vi "Main.vi"() -> ()   [LabVIEW 2020]
uses:
  Global_Variable/Global.vi
  Database/Global1.vi
  <userlib>/_MGI/Menu Building/MenuTypes/MenuStrip/MGI_MenuStrip.lvclass
  Libraries/S7/S7.lvlib
  <userlib>/_MGI/Menu Building/MenuItemStatusChange/MGI_MenuItemStatusChange.lvclass
  System.Windows.Forms
panel:
  in  "VI引用句柄":refnum<vi>
  out "结果显示:":string
  out "传感器值":dbl format="%#_4gN"
  in  "打印条码":bool caption="布尔"
  out "自动":bool
  out "管柱码":string
  out "上序状态":string
  in  "Andon":enum32{"未选择", "缺料报警", "质量报警", "故障报警"}(radio)
  out "PLC":bool
  in  "菜单":refnum<k24>(container)
  in  "Result":string[][](table)
  out "试验计时":u16 format="%.0fS"
  out "生产数量":i32 format="%.0f件"
  out "合格数量":i32 format="%.0f件"
  out "userStatus":string caption="用户状态"
  out "userName":string caption="用户名"
  out "connectionMode":string caption="联机类型"
  out "产品型号":string
  out "锁紧/开启":bool
  out "提示信息":string
  out "错误":bool
  out "时间字符串":string
  out "日期字符串":string
  # "中间轴装配"
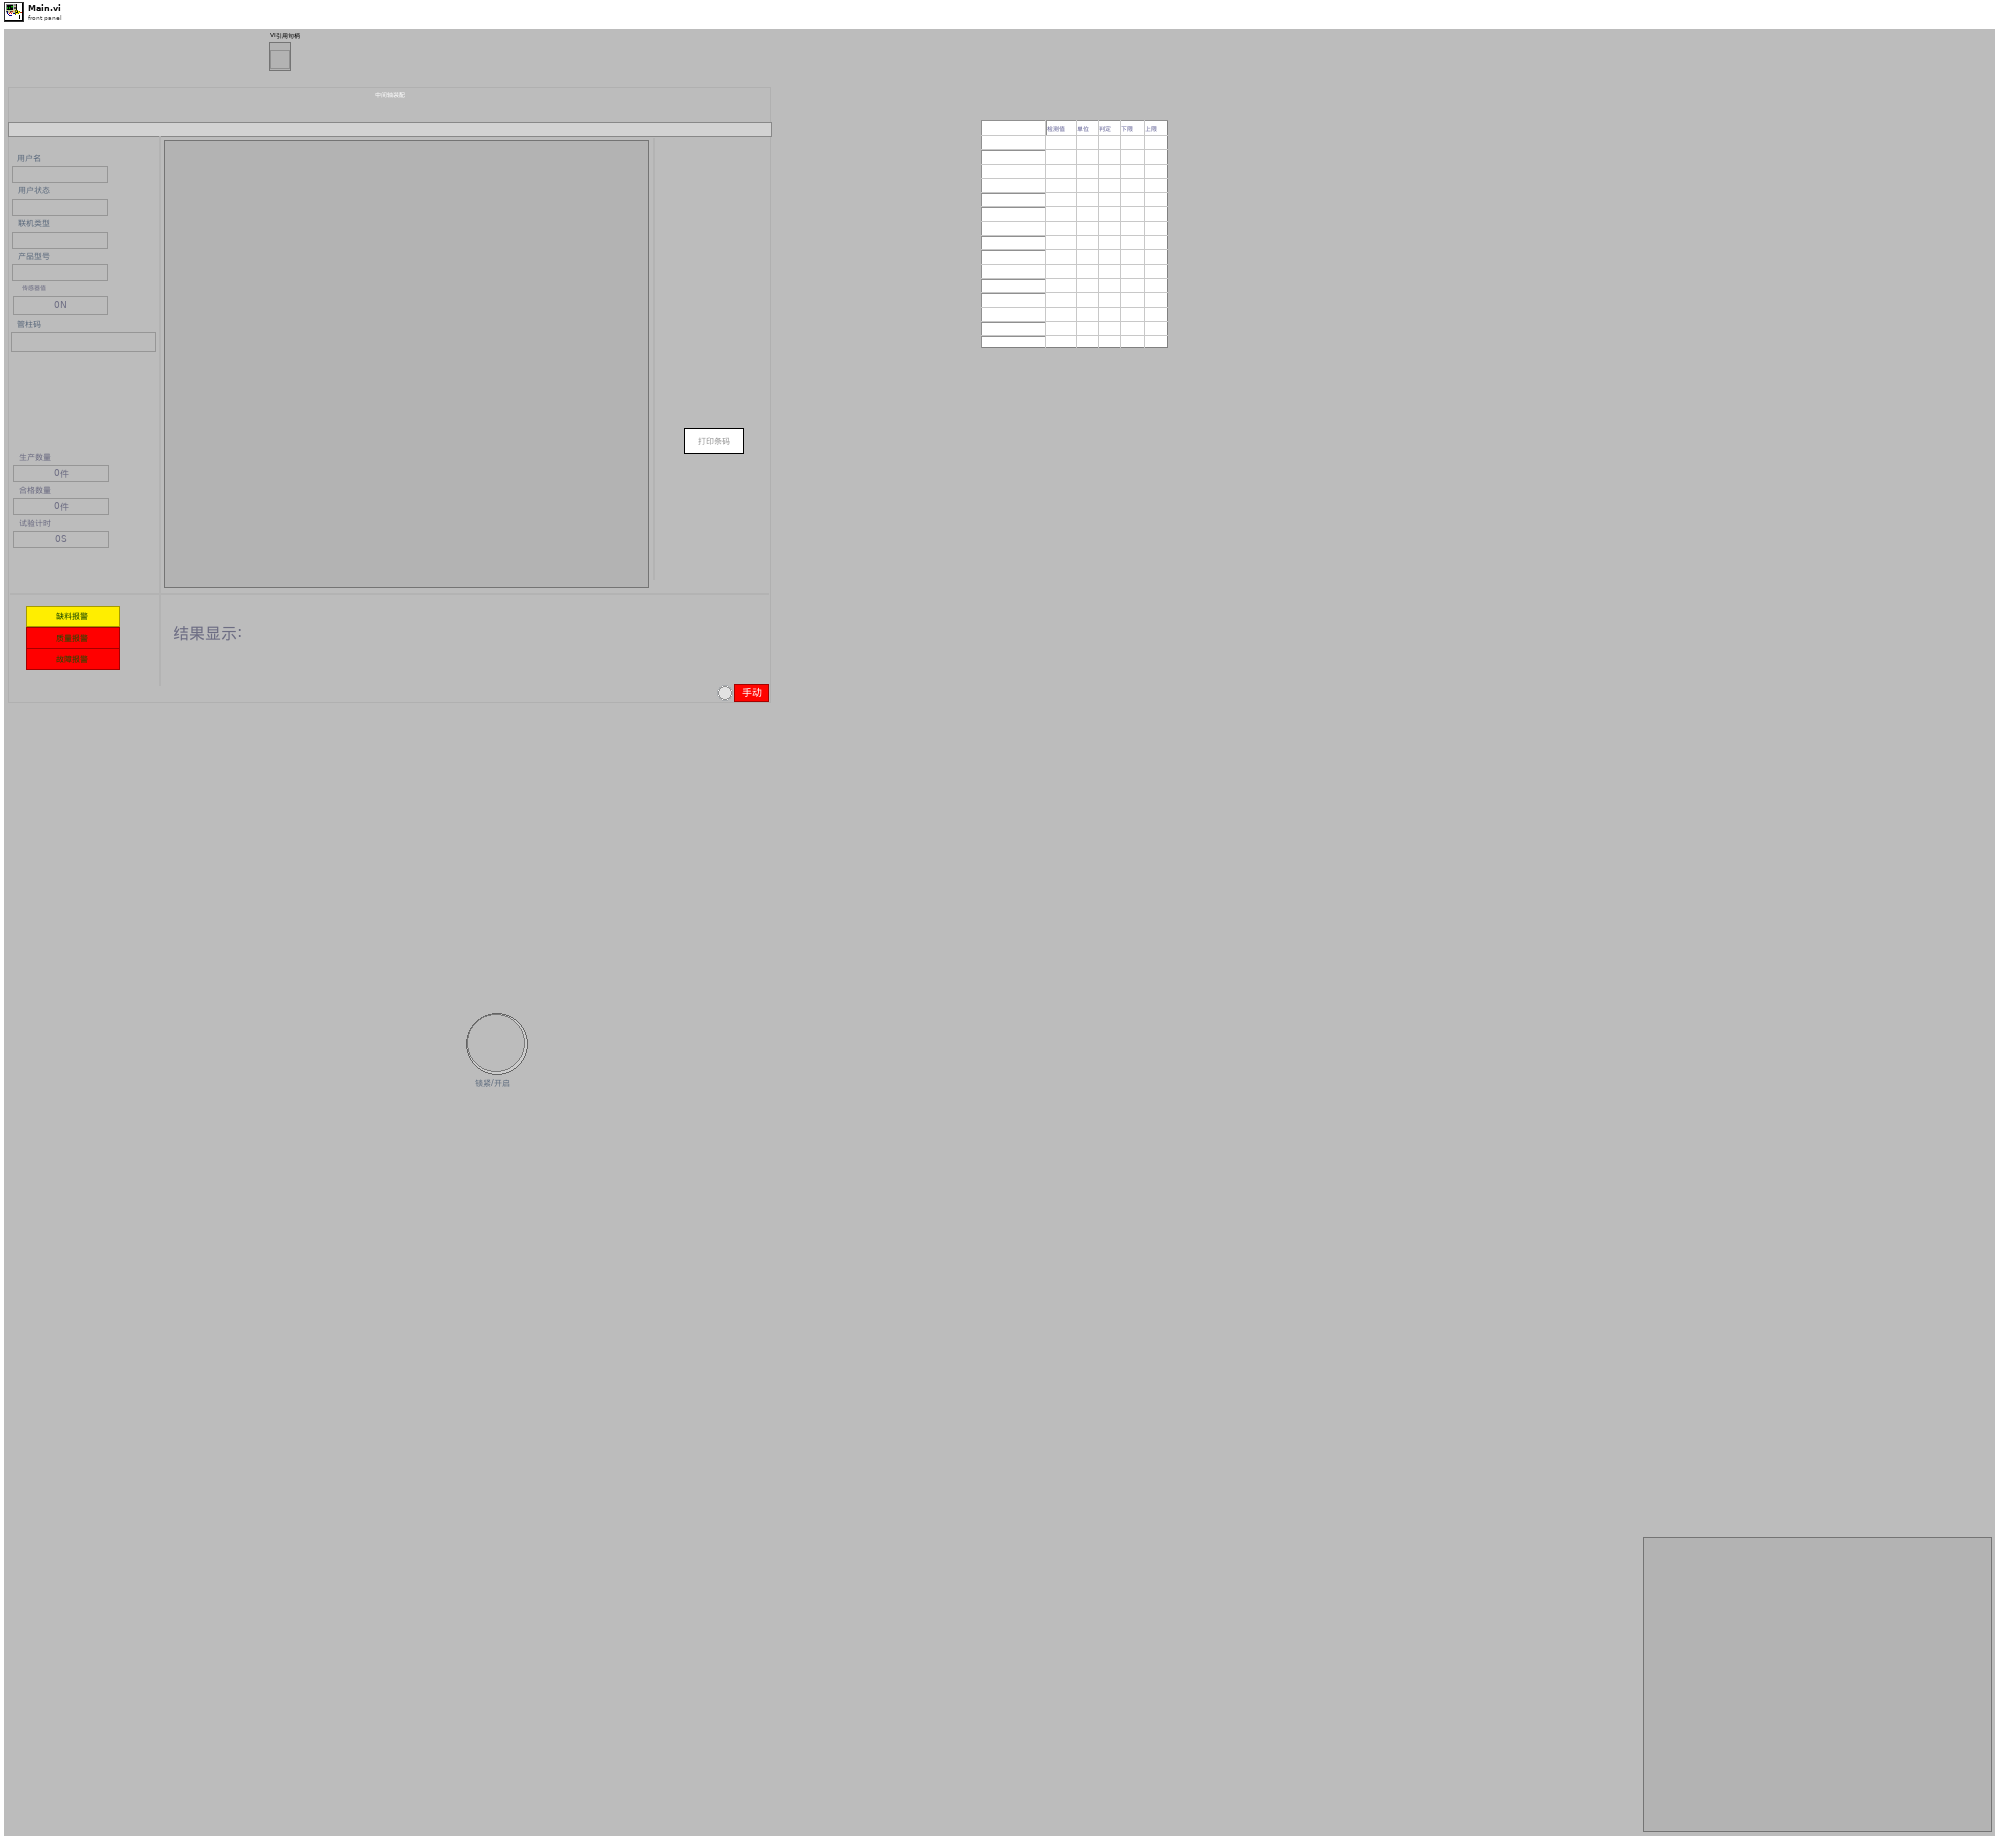
[diagram p1: front panel]
types:
  T1 = typedef "S7.lvlib/Broadcast Events--cluster.ctl" = cluster{"Module Did Init":refnum<user-event>, "Status Updated":refnum<user-event>, "Error Reported":refnum<user-event>, "Module Did Stop":refnum<user-event>, "Update Module Execution Status":refnum<user-event>}
  T2 = enum32{"Invalid", "Standard", "Closed", "Hidden", "Minimized", "Maximized"}
  T3 = cluster{"设备名称":string, "操作人员":string, "设备状态":enum16{"设备离线", "设备正常", "设备缺料", "设备故障", "质量报警"}, "附加信息":string}
  T4 = enum32{"invalid app kind", "Development System", "Run Time System", "Student Edition", "Embedded LabVIEW", "Evaluation", "Custom"}
  T5 = cluster{"扭矩":sgl, "输入移载位移":sgl, "工装移载位移":sgl, "输入编码位移":sgl, "输入扭矩":sgl, "输出扭矩(小)":sgl, "输出扭矩(大)":sgl, "吸收电流":sgl}
  T6 = cluster{"用户编号":string, "用户名":string, "用户密码(密文)":string, "用户权限":string}
  T7 = cluster{"Core":cluster{"Current VI Reference":refnum<vi>, "Close Panel on Exit?":bool}, "Your Boolean data":bool, "Your string data":string}
  T8 = enum32{"Bad", "Idle", "Run top level", "Running"}
  T9 = cluster{"Current VI Reference":refnum<vi>, "Close Panel on Exit?":bool}
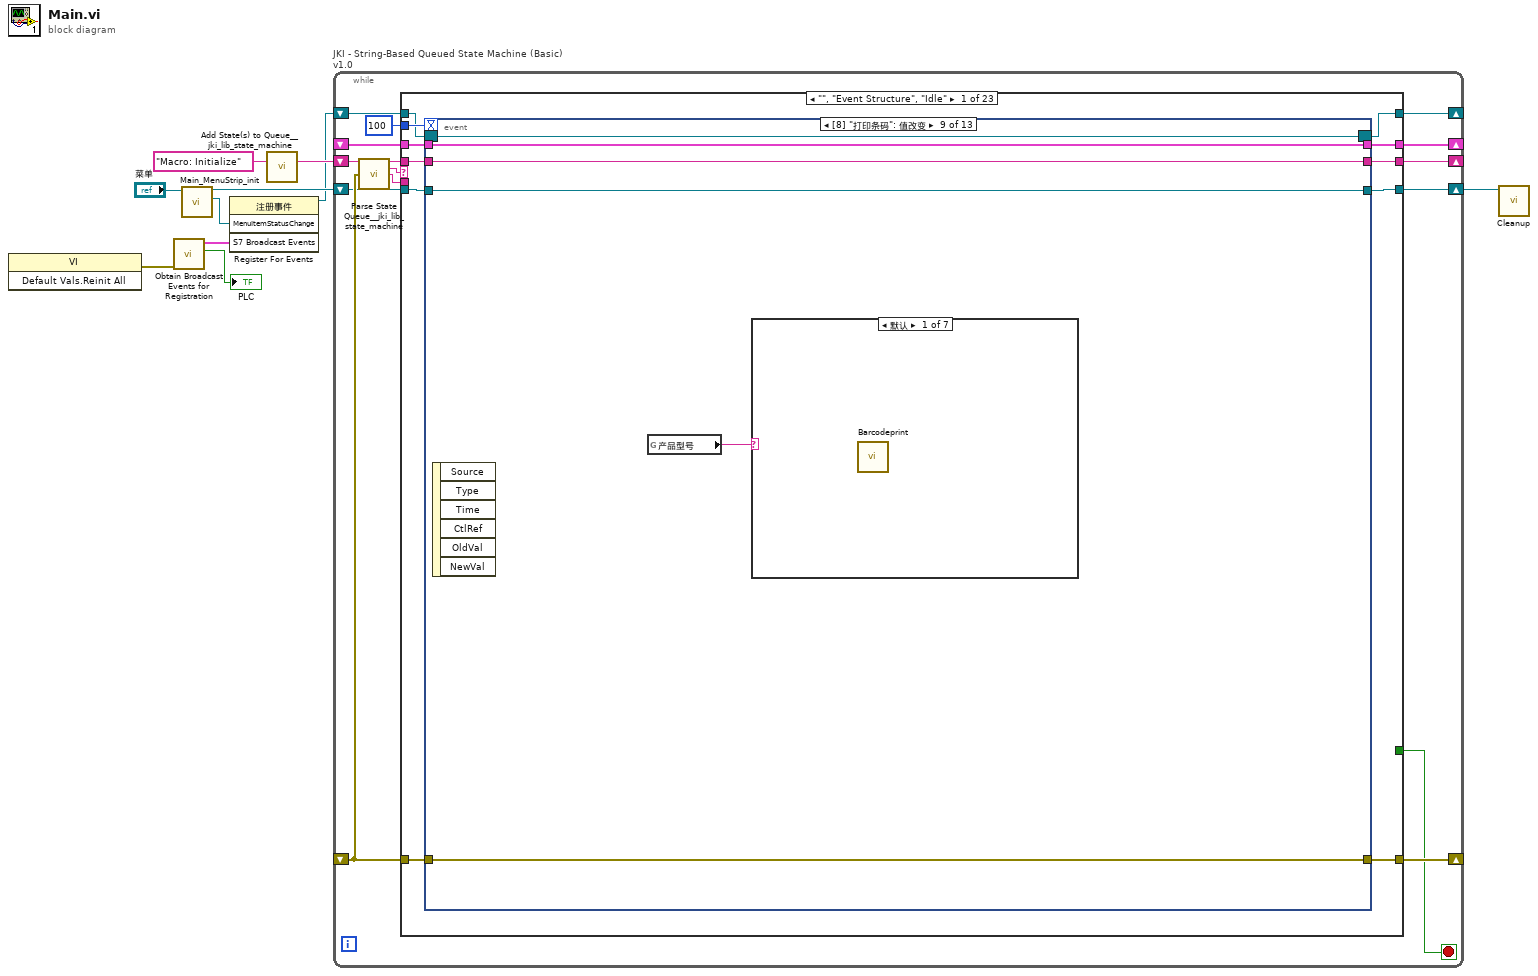
[diagram p0: block diagram]
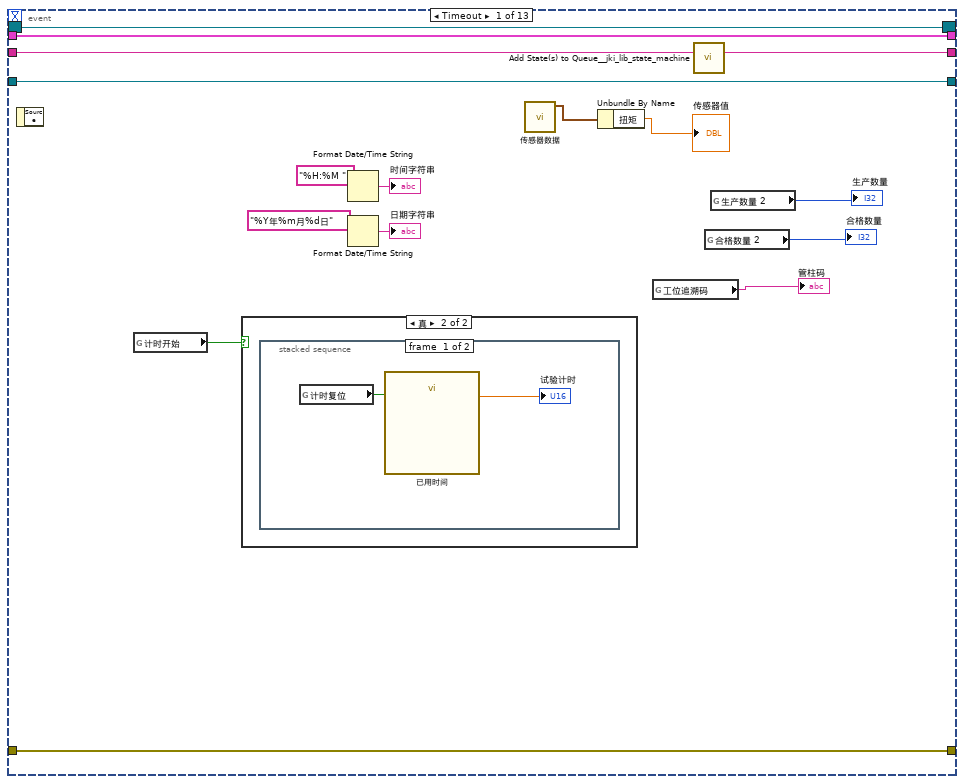
[diagram p2: hidden frame]
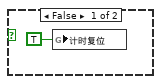
[diagram p3: hidden frame]
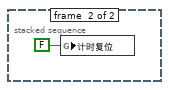
[diagram p4: hidden frame]
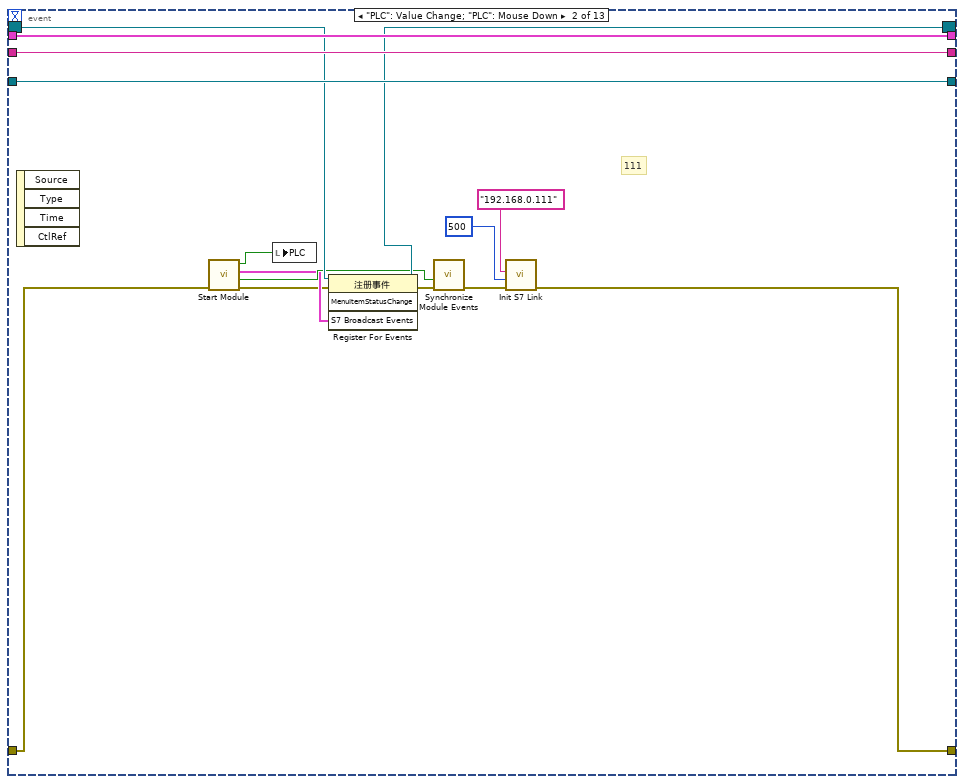
[diagram p5: hidden frame]
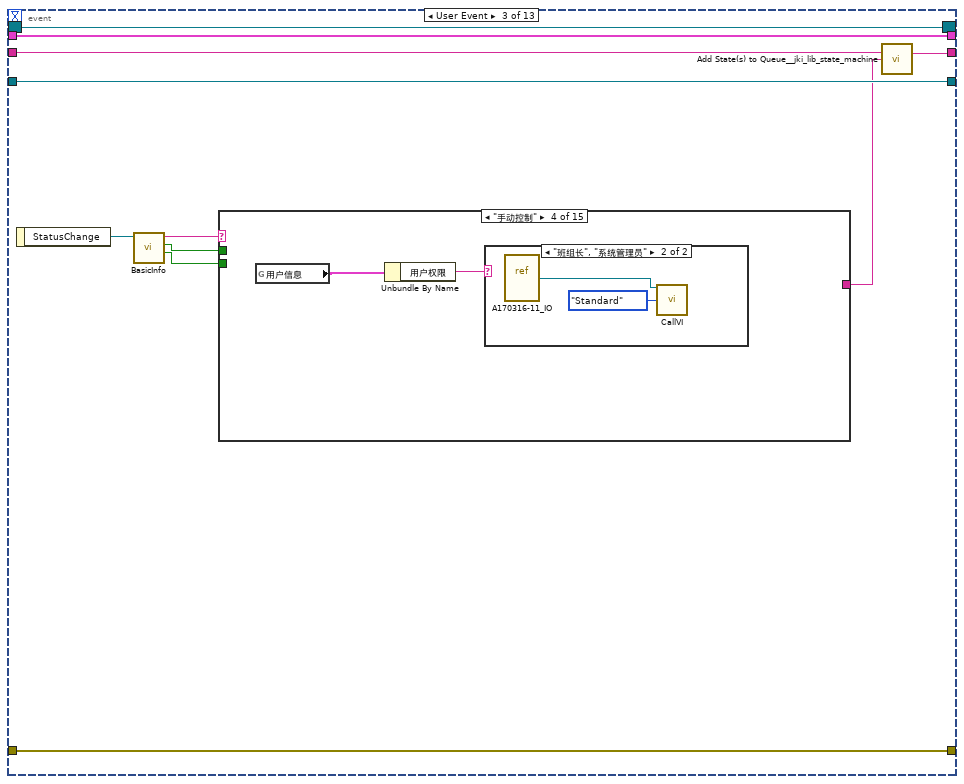
[diagram p6: hidden frame]
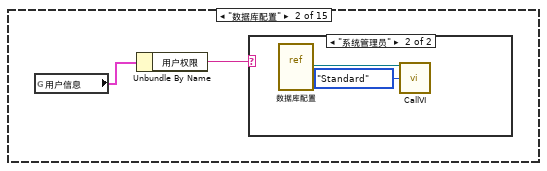
[diagram p8: hidden frame]
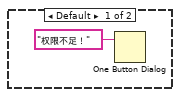
[diagram p9: hidden frame]
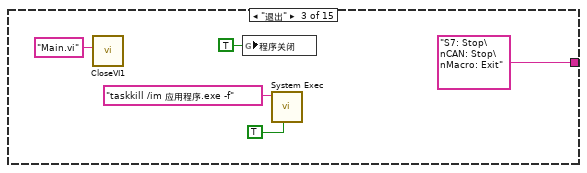
[diagram p10: hidden frame]
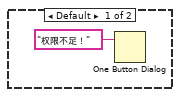
[diagram p11: hidden frame]
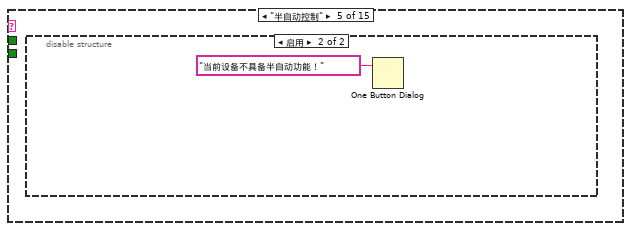
[diagram p12: hidden frame]
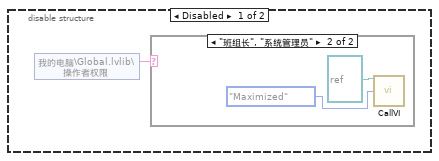
[diagram p13: hidden frame]
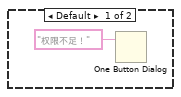
[diagram p14: hidden frame]
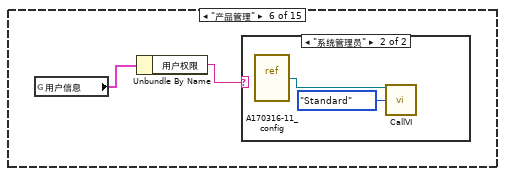
[diagram p15: hidden frame]
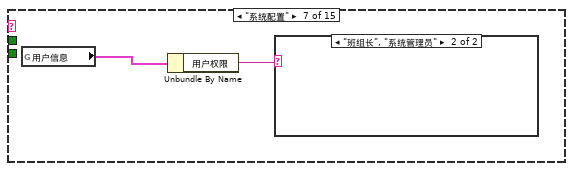
[diagram p17: hidden frame]
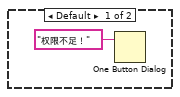
[diagram p18: hidden frame]
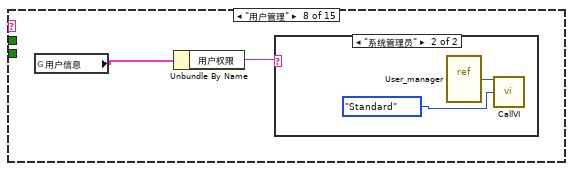
[diagram p19: hidden frame]
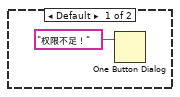
[diagram p20: hidden frame]
diagram:
  n1 = invoke class="VI" method="Default Vals.Reinit All"() -> (error out=w3:errorcluster)  [unwired: 3 in, 2 out]
  n2 = call "Obtain Broadcast Events for Registration.vi"("error in (no error)"=w3) -> ("Already running?"=→"PLC":bool, "S7 Broadcast Events"=w5:T1)  [unwired: 8 in, 1 out]
  n3 = call "Main_MenuStrip_init.vi"("MenuStrip"="菜单") -> ("MenuItemStatusChange"=w2:refnum<user-event>, "Menu out"=w7:refnum<class "MGI_MenuStrip.lvclass">)  [unwired: 9 in]
  n4 = register-events(w2, w5) -> (reference out=w1:refnum<event-registration>)  [unwired: 2 in, 1 out]
  n5 = call <vilib>:"Add State(s) to Queue__jki_lib_state_machine.vi"("State(s) in (\"\")"="Macro: Initialize") -> ("States Out"=w10:string)  [unwired: 14 in]
  n6 = while "JKI - String-Based Queued State Machine (Basic) v1.0" {
    shift-right: [w19] -> _
    shift-left: _ -> [w18]
    shift-right: [w21] -> _
    shift-left: _ -> [w16]
    shift-right: [w20] -> _
    shift-left: w10 -> [w22]
    shift-right: [w14] -> w6
    shift-left: w7 -> [w15]
    shift-right: [w12] -> _
    shift-left: w1 -> [w11]
    stop <- w13 stop-if-true
    n7 = call <vilib>:"Parse State Queue__jki_lib_state_machine.vi"("State Queue"=w22, "Error In (no error)"=w16) -> ("Remaining States"=w24:string, "Current State"=w25:string, "Arguments"=w23:string)  [unwired: 11 in]
    n8 = case shown="\"\", \"Event Structure\", \"Idle\"" w25 {
      selector: w25 -> [_ _ w240 _ _ _ _ _ _ _ _ _ _ _ _ _ _ _ _ _ _ _ _]
      tunnel: w24 -> [w36 w237 w244 w264 w272 w279 w285 w289 w295 w301 w322 w331 w342 w350 w356 w363 w390 w419 w427 w440 w468 w475 w492]
      tunnel: w23 -> [_ _ _ _ _ _ _ _ _ _ _ _ _ _ _ _ _ _ w422 w434 _ _ _]
      tunnel: w18 -> [w34 w234 w242 w255 w269 w277 w282 w290 w298 w304 w325 w328 _ w345 w353 w361 w388 w416 w425 w436 w465 w472 w489]
      tunnel: [w33 w235 w246 w261 errorcluster {"status"=FALSE, "code"=0, "source"=""} ("error out") w276 w283 w287 w293 w300 w321 w329 w339 w346 w354 w360 w386 w417 w423 w437 w466 w473 w490] -> w21
      tunnel: w16 -> [w32 w235 w245 w261 w268 w276 w283 w287 w294 w300 w321 w329 w339 w347 w354 w357 w386 w417 w424 w438 w466 w473 w490]
      tunnel: [w35 w236 w243 w263 w271 w278 w284 w289 w296 w302 w323 w330 w341 w349 w355 w362 w389 w418 w426 w439 w467 w474 w491] -> w20
      tunnel: [w31 w234 w242 w262 w269 w277 w282 w290 w298 w304 w325 w328 w340 w345 w353 w361 w388 w416 w425 w436 w465 w472 w489] -> w19
      tunnel: 100 ("Timeout") -> [w30 _ _ _ _ _ _ _ _ _ _ _ _ _ _ _ _ _ _ _ _ _ _]
      tunnel: w15 -> [w29 w233 w239 w252 w266 w275 w281 w288 w297 w303 w324 w327 w333 w344 w352 w359 w387 w415 w421 w433 w464 w470 w482]
      tunnel: [w28 w233 w239 w252 w266 w275 w281 w288 w297 w303 w324 w327 w333 w344 w352 w359 w387 w415 w421 w433 w464 w470 w482] -> w14
      tunnel: [_ _ _ _ _ TRUE _ _ _ _ _ _ _ _ _ _ _ _ _ _ _ _ _] -> w13
      tunnel: [w26 w232 w238 w251 w265 w273 w280 w291 w292 w299 w320 w326 w334 w343 w351 w358 w385 w414 w420 w432 w463 w469 w481] -> w12
      tunnel: w11 -> [w27 w232 w238 w251 w265 w273 w280 w291 w292 w299 w320 w326 w334 w343 w351 w358 w385 w414 w420 w432 w463 w469 w481]
      frame "", "Event Structure", "Idle" {
        n9 = event shown="[8] \"打印条码\": 值改变" {
          selector: w27 -> [w43 w66 w72 w137 w144 w151 w158 w173 w187 w190 w195 w206 _]
          dyn-events: [w43 w65 w72 w137 w144 w151 w158 w173 w187 w190 w195 w206 _] -> w26
          timeout: w30 -> [_ _ _ _ _ _ _ _ _ _ _ _ _]
          tunnel: w36 -> [w52 w70 w81 w138 w145 w154 w161 w170 w186 w192 w202 w208 w226]
          tunnel: [w51 w70 w79 w139 w146 w155 w162 w171 w186 w193 w201 w209 w226] -> w35
          tunnel: w34 -> [w50 w71 w80 w141 w149 w156 w163 w172 w188 w194 w199 w203 w227]
          tunnel: [w44 w67 w82 w142 w147 w152 w164 w168 w184 w191 w200 w210 w224] -> w33
          tunnel: w32 -> [w44 w68 w82 w142 w147 w152 w165 w168 w184 w191 w200 w210 w224]
          tunnel: [w50 w71 w80 w141 w149 w156 w163 w172 w188 w194 w199 w203 w227] -> w31
          tunnel: w29 -> [w42 w69 w75 w140 w148 w153 w160 w169 w185 _ _ w204 w225]
          tunnel: [w42 w69 w75 w140 w148 w153 w160 w169 w185 _ _ w204 w225] -> w28
          event Timeout {
            n10 = event-data() -> ()  [unwired: 1 in, 1 out]
            n11 = global read "Global.vi" "计时开始"() -> (w45:bool)
            n12 = case shown="真" w45 {
              frame False {
                n13 = global write "Global.vi" "计时复位"(TRUE ("计时复位")) -> ()
              }
              frame True {
                n14 = stacked-sequence {
                  frame #0 {
                    n15 = global read "Global.vi" "计时复位"() -> (w54:bool)
                    n16 = call "已用时间"("Reset"=w54) -> ("Elapsed Time (s)"=→"试验计时":dbl)  [unwired: 11 in, 7 out]
                  }
                  frame #1 {
                    n17 = global write "Global.vi" "计时复位"(FALSE ("计时复位")) -> ()
                  }
                }
              }
            }
            n18 = Format Date/Time String(time format string (%c)="%H:%M ") -> (date/time string=→"时间字符串":string)  [unwired: 2 in]
            n19 = Format Date/Time String(time format string (%c)="%Y年%m月%d日") -> (date/time string=→"日期字符串":string)  [unwired: 2 in]
            n20 = call "传感器数据.vi"() -> ("传感器读数"=w39:T5)  [unwired: 11 in]
            n21 = Unbundle By Name(w39) -> ("扭矩"=→"传感器值":sgl)
            n22 = global read "Global1.vi" "工位追溯码"() -> (→"管柱码":string)
            n23 = call <vilib>:"Add State(s) to Queue__jki_lib_state_machine.vi"("State(s) in (\"\")"=w52) -> ("States Out"=w51:string)  [unwired: 14 in]
            n24 = global read "Global.vi" "合格数量 2"() -> (→"合格数量":i32)
            n25 = global read "Global.vi" "生产数量 2"() -> (→"生产数量":i32)
          }
          event "PLC": Value Change; "PLC": Mouse Down {
            # "111"
            n26 = event-data() -> ()  [unwired: 1 in, 4 out]
            n27 = call "Start Module.vi"("error in (no error)"=w68) -> ("error out"=w61:errorcluster, "Wait for Event Sync?"=w64:bool, "S7 Broadcast Events"=w63:T1, "Module Was Already Running?"=w62:bool)  [unwired: 7 in]
            n28 = local write "PLC"(w62) -> ()
            n29 = register-events(reference=w66, error in=w61, w63) -> (reference out=w65:refnum<event-registration>, error out=w60:errorcluster)  [unwired: 1 in]
            n30 = call "Synchronize Module Events.vi"("error in (no error)"=w60, "Wait for Event Sync?"=w64) -> ("error out"=w59:errorcluster)  [unwired: 9 in]
            n31 = call "Init S7 Link.vi"("error in (no error)"=w59, "超时"=500, "IP"="192.168.0.111") -> ("error out"=w67:errorcluster)  [unwired: 8 in]
          }
          event User Event {
            n32 = event-data() -> ("StatusChange"=w73:refnum<class "MGI_MenuItemStatusChange.lvclass">)  [unwired: 1 in]
            n33 = call <userlib>:"BasicInfo.vi"("MGI_MenuItemStatusChange in"=w73) -> ("Enabled?"=w76:bool, "Checked?"=w77:bool, "Tag"=w78:string)  [unwired: 7 in, 1 out]
            n34 = case shown="\"手动控制\"" w78 {
              tunnel: w77 -> [_ _ _ _ _ _ _ _ _ _ _ _ _ _ _]
              tunnel: w76 -> [_ _ _ _ _ _ _ _ _ _ _ _ _ _ _]
              tunnel: [_ _ "S7: Stop\nCAN: Stop\nMacro: Exit" _ _ _ _ _ _ _ _ _ _ _ _] -> w74
              frame "假", Default {
              }
              frame "数据库配置" {
                n35 = global read "Global1.vi" "用户信息"() -> (w83:T6)
                n36 = Unbundle By Name(w83) -> ("用户权限"=w84:string)
                n37 = case shown="\"系统管理员\"" w84 {
                  frame Default {
                    n38 = One Button Dialog(message="权限不足！" ("消息")) -> ()  [unwired: 1 in, 1 out]
                  }
                  frame "系统管理员" {
                    n39 = vi-ref "数据库配置.vi"() -> (w86:refnum<vi>)
                    n40 = call "CallVI.vi"("VI引用"=w86, "状态"=T2."Standard") -> ()  [unwired: 11 in, 3 out]
                  }
                }
              }
              frame "退出" {
                n41 = call "CloseVI1.vi"("名称或相对路径"="Main.vi") -> ()  [unwired: 10 in, 1 out]
                n42 = global write "Global.vi" "程序关闭"(TRUE ("程序关闭")) -> ()
                n43 = call <vilib>:"System Exec.vi"("run minimized? (F)"=TRUE, "command line"="taskkill /im 应用程序.exe -f") -> ()  [unwired: 6 in, 4 out]
              }
              frame "手动控制" {
                n44 = global read "Global1.vi" "用户信息"() -> (w93:T6)
                n45 = Unbundle By Name(w93) -> ("用户权限"=w94:string)
                n46 = case shown="\"班组长\", \"系统管理员\"" w94 {
                  frame Default {
                    n47 = One Button Dialog(message="权限不足！" ("消息")) -> ()  [unwired: 1 in, 1 out]
                  }
                  frame "班组长", "系统管理员" {
                    n48 = vi-ref "A170316-11_IO.vi"() -> (w96:refnum<vi>)
                    n49 = call "CallVI.vi"("VI引用"=w96, "状态"=T2."Standard") -> ()  [unwired: 11 in, 3 out]
                  }
                }
              }
              frame "半自动控制" {
                n50 = disable-structure shown="启用" {
                  frame Disabled {
                    n51 = shared-variable "我的电脑\\Global.lvlib\\操作者权限"() -> (w98:string)  [unwired: 1 in, 1 out]
                    n52 = case shown="\"班组长\", \"系统管理员\"" w98 {
                      frame Default {
                        n53 = One Button Dialog(message="权限不足！" ("消息")) -> ()  [unwired: 1 in, 1 out]
                      }
                      frame "班组长", "系统管理员" {
                        n54 = call "CallVI.vi"("VI引用"=refnum<vi> refnum, "状态"=T2."Maximized") -> ()  [unwired: 11 in, 3 out]
                      }
                    }
                  }
                  frame Enabled {
                    n55 = One Button Dialog(message="当前设备不具备半自动功能！" ("消息")) -> ()  [unwired: 1 in, 1 out]
                  }
                }
              }
              frame "产品管理" {
                n56 = global read "Global1.vi" "用户信息"() -> (w104:T6)
                n57 = Unbundle By Name(w104) -> ("用户权限"=w103:string)
                n58 = case shown="\"系统管理员\"" w103 {
                  frame "假", Default {
                  }
                  frame "系统管理员" {
                    n59 = vi-ref "A170316-11_config.vi"() -> (w106:refnum<vi>)
                    n60 = call "CallVI.vi"("VI引用"=w106, "状态"=T2."Standard") -> ()  [unwired: 11 in, 3 out]
                  }
                }
              }
              frame "系统配置" {
                n61 = global read "Global1.vi" "用户信息"() -> (w107:T6)
                n62 = Unbundle By Name(w107) -> ("用户权限"=w108:string)
                n63 = case shown="\"班组长\", \"系统管理员\"" w108 {
                  frame Default {
                    n64 = One Button Dialog(message="权限不足！" ("消息")) -> ()  [unwired: 1 in, 1 out]
                  }
                  frame "班组长", "系统管理员" {
                  }
                }
              }
              frame "用户管理" {
                n65 = global read "Global1.vi" "用户信息"() -> (w110:T6)
                n66 = Unbundle By Name(w110) -> ("用户权限"=w111:string)
                n67 = case shown="\"系统管理员\"" w111 {
                  frame Default {
                    n68 = One Button Dialog(message="权限不足！" ("消息")) -> ()  [unwired: 1 in, 1 out]
                  }
                  frame "系统管理员" {
                    n69 = vi-ref "User_manager.vi"() -> (w114:refnum<vi>)
                    n70 = call "CallVI.vi"("VI引用"=w114, "状态"=T2."Standard") -> ()  [unwired: 11 in, 3 out]
                  }
                }
              }
              frame "编码规则" {
                n71 = global read "Global1.vi" "用户信息"() -> (w115:T6)
                n72 = Unbundle By Name(w115) -> ("用户权限"=w116:string)
                n73 = case shown="\"班组长\", \"工艺管理员\", \"系统管理员\"" w116 {
                  frame Default {
                    n74 = One Button Dialog(message="权限不足！" ("消息")) -> ()  [unwired: 1 in, 1 out]
                  }
                  frame "班组长", "工艺管理员", "系统管理员" {
                    n75 = vi-ref "编码规则设置.vi"() -> (w119:refnum<vi>)
                    n76 = call "CallVI.vi"("VI引用"=w119, "状态"=T2."Standard") -> ()  [unwired: 11 in, 3 out]
                  }
                }
              }
              frame "易损件管理" {
                n77 = vi-ref "易损件管理.vi"() -> (w121:refnum<vi>)
                n78 = call "CallVI.vi"("VI引用"=w121, "状态"=T2."Standard") -> ()  [unwired: 11 in, 3 out]
              }
              frame "物料批次管理" {
                n79 = vi-ref "批次管理.vi"() -> (w123:refnum<vi>)
                n80 = call "CallVI.vi"("VI引用"=w123, "状态"=T2."Standard") -> ()  [unwired: 11 in, 3 out]
              }
              frame "报表" {
                n81 = call "文件对话框"("start path"=path "D:/report", "prompt"="打开报表", "pattern (all files)"="*.doc;*.docx", "pattern label"="Word 文档") -> ("selected path"=w124:path, "error out"=w125:errorcluster)  [unwired: 8 in, 2 out]
                n82 = case shown="无错误" w125 {
                  selector: w125 -> [w131 w133]
                  tunnel: w124 -> [w132 _]
                  frame No Error {
                    w130 = 1 items=["Normal", "Maximize", "Minimize"] ("cpubbs_WindowState")
                    n83 = call "Open_Word.vi"("File Path"=w132, "cpubbs_WindowState"=w130, "错误输入（无错误）"=w131) -> ()  [unwired: 12 in, 1 out]
                  }
                  frame Error {
                    n84 = call <vilib>:"Clear Errors.vi"("error in (no error)"=w133) -> ()  [unwired: 5 in, 2 out]
                  }
                }
              }
              frame "报警信息" {
              }
              frame "关于" {
              }
              frame "操作演示" {
                n85 = call <vilib>:"Application Directory.vi"() -> ("Application Directory"=w136:path)
                n86 = Build Path(base path=w136, name or relative path="操作演示" ("名称或相对路径")) -> (appended path=w135:path)
                n87 = call "自动播放ppt.vi"("路径"=w135) -> ()  [unwired: 10 in, 1 out]
              }
            }
            n88 = call <vilib>:"Add State(s) to Queue__jki_lib_state_machine.vi"("State(s) in (\"\")"=w81, "State(s) at Back (\"\")"=w74) -> ("States Out"=w79:string)  [unwired: 13 in]
          }
          event User Event {
            n89 = event-data() -> ("Init?"=w143:bool)  [unwired: 1 in, 1 out]
            n90 = local write "PLC"(w143) -> ()
            n91 = call <vilib>:"Add State(s) to Queue__jki_lib_state_machine.vi"("State(s) in (\"\")"=w138) -> ("States Out"=w139:string)  [unwired: 14 in]
          }
          event User Event {
            n92 = event-data() -> ("Running?"=w150:bool)  [unwired: 1 in]
            n93 = local write "PLC"(w150) -> ()
            n94 = call <vilib>:"Add State(s) to Queue__jki_lib_state_machine.vi"("State(s) in (\"\")"=w145) -> ("States Out"=w146:string)  [unwired: 14 in]
          }
          event User Event {
            n95 = event-data() -> ()  [unwired: 1 in, 7 out]
            n96 = local write "PLC"(FALSE ("PLC")) -> ()
            n97 = call <vilib>:"Add State(s) to Queue__jki_lib_state_machine.vi"("State(s) in (\"\")"=w154) -> ("States Out"=w155:string)  [unwired: 14 in]
          }
          event User Event {
            n98 = event-data() -> ("Error"=w166:errorcluster)  [unwired: 1 in]
            n99 = Merge Errors(w166, w165) -> (w164:errorcluster)
            n100 = call <vilib>:"Add State(s) to Queue__jki_lib_state_machine.vi"("State(s) in Front (\"\")"="S7: Initialize\nIdle", "State(s) in (\"\")"=w161) -> ("States Out"=w162:string)  [unwired: 13 in]
          }
          event "自动": Mouse Down {
            n101 = event-data() -> ()  [unwired: 1 in, 8 out]
            n102 = local read "自动"() -> (w167:bool)
            n103 = case shown="假" w167 {
              frame False {
                n104 = global read "Global.vi" "设备状态"() -> (w174:i32)
                n105 = case shown="5" w174 {
                  frame 0, Default {
                    n106 = One Button Dialog(message="请复位！" ("消息")) -> ()  [unwired: 1 in, 1 out]
                  }
                  frame 5 {
                    n107 = vi-ref "A170316-11_Auto.vi"() -> (w178:refnum<vi>)
                    n108 = invoke class="VI" method="Ctrl Val.Set"(reference=w178, "Control Name"="STEP" ("控件名"), "Value"="初始化" ("控件名")) -> ()  [unwired: 2 in, 5 out]
                  }
                }
              }
              frame True {
                n109 = Two Button Dialog(message="确定要退出自动？" ("消息")) -> (T button?=w179:bool)  [unwired: 2 in]
                n110 = case shown="真" w179 {
                  frame False {
                  }
                  frame True {
                    n111 = vi-ref "A170316-11_Auto.vi"() -> (w183:refnum<vi>)
                    n112 = invoke class="VI" method="Ctrl Val.Set"(reference=w183, "Control Name"="STEP" ("控件名"), "Value"="手动" ("控件名")) -> ()  [unwired: 2 in, 5 out]
                  }
                }
              }
            }
            n113 = call <vilib>:"Add State(s) to Queue__jki_lib_state_machine.vi"("State(s) in (\"\")"=w170) -> ("States Out"=w171:string)  [unwired: 14 in]
          }
          event "打印条码": Value Change {
            n114 = event-data() -> ()  [unwired: 1 in, 6 out]
            n115 = global read "Global.vi" "产品型号"() -> (w189:string)
            n116 = case shown="默认" w189 {
              frame Default {
                n117 = call "Barcodeprint.vi"() -> ()  [unwired: 12 in]
              }
              frame "R92A" {
                n118 = call "BarcodeprintR92A.vi"() -> ()  [unwired: 12 in]
              }
              frame "R092B" {
                n119 = call "BarcodeprintR92A.vi"() -> ()  [unwired: 12 in]
              }
              frame "R092C" {
                n120 = call "BarcodeprintR92A.vi"() -> ()  [unwired: 12 in]
              }
              frame "R092D" {
                n121 = call "BarcodeprintR92A.vi"() -> ()  [unwired: 12 in]
              }
              frame "R567B" {
                n122 = call "BarcodeprintR92A.vi"() -> ()  [unwired: 12 in]
              }
              frame "R567D" {
                n123 = call "BarcodeprintR92A.vi"() -> ()  [unwired: 12 in]
              }
            }
          }
          event "错误": Mouse Down {
            n124 = event-data() -> ()  [unwired: 1 in, 8 out]
            n125 = call <vilib>:"Add State(s) to Queue__jki_lib_state_machine.vi"("State(s) in (\"\")"=w192) -> ("States Out"=w193:string)  [unwired: 14 in]
          }
          event Panel Close? {
            n126 = event-data() -> ()  [unwired: 1 in, 1 out]
            n127 = global write "Global.vi" "程序关闭"(TRUE ("程序关闭")) -> ()
            n128 = call <vilib>:"Add State(s) to Queue__jki_lib_state_machine.vi"("State(s) in Front (\"\")"="S7: Stop\nMacro: Exit", "State(s) in (\"\")"=w202) -> ("States Out"=w201:string)  [unwired: 13 in]
            n129 = event-data("Discard?"=TRUE) -> ()  [unwired: 1 in, 1 out]
          }
          event "VI引用句柄": Value Change {
            n130 = event-data() -> ("NewVal"=w207:refnum<vi>)  [unwired: 1 in, 5 out]
            n131 = stacked-sequence {
              tunnel: w207 -> [w211 _ _]
              tunnel: [_ _ w215] -> w205
              frame #0 {
                n132 = disable-structure shown="禁用" {
                  disable-tunnel: w211 -> [w213 _]
                  frame Disabled {
                    n133 = control-ref of="子面板"() -> (w212:refnum<vi>)
                    n134 = call "Call_SubPanal.vi"("VI引用句柄"=w213, "SubPnl引用句柄"=w212) -> ()  [unwired: 9 in, 1 out]
                  }
                  frame Enabled {
                  }
                }
              }
              frame #1 {
                n135 = global read "Global.vi" "产品型号"() -> (w214:string)
                n136 = local write "产品型号"(w214) -> ()
              }
              frame #2 {
                n137 = global read "Global.vi" "启用CAN"() -> (w216:bool)
                n138 = case shown="真" w216 {
                  tunnel: ["CAN: Stop" "CAN: Stop\nIdle\nCAN: Start"] -> w215
                  frame False {
                  }
                  frame True {
                  }
                }
              }
            }
            n139 = call <vilib>:"Add State(s) to Queue__jki_lib_state_machine.vi"("State(s) in Front (\"\")"=w205, "State(s) in (\"\")"=w208) -> ("States Out"=w209:string)  [unwired: 13 in]
          }
          event "Andon": Value Change {
            n140 = event-data() -> ("NewVal"=w223:enum32{"未选择", "缺料报警", "质量报警", "故障报警"})  [unwired: 1 in]
            n141 = case shown="\"质量报警\"" w223 {
              tunnel: [enum16{"设备离线", "设备正常", "设备缺料", "设备故障", "质量报警"}."设备正常" ("设备状态") enum16{"设备离线", "设备正常", "设备缺料", "设备故障", "质量报警"}."设备缺料" ("设备状态") enum16{"设备离线", "设备正常", "设备缺料", "设备故障", "质量报警"}."质量报警" ("设备状态") enum16{"设备离线", "设备正常", "设备缺料", "设备故障", "质量报警"}."设备故障" ("设备状态")] -> w221
              frame "未选择", Default {
              }
              frame "缺料报警" {
              }
              frame "质量报警" {
              }
              frame "故障报警" {
              }
            }
            n142 = local read "userName"() -> (w220:string)
            n143 = Bundle By Name(cluster=T3 {"设备名称"="中间轴装配", "操作人员"="", "设备状态"=enum."设备离线", "附加信息"=""} ("设备信息"), "操作人员"=w220, "设备状态"=w221) -> (w219:T3)
            n144 = call "Change_Client.vi"("设备信息"=w219) -> ()  [unwired: 10 in, 1 out]
          }
        }
      }
      frame "---------- Core ----------" {
        n145 = call <vilib>:"Add State(s) to Queue__jki_lib_state_machine.vi"("State(s) in (\"\")"=w237) -> ("States Out"=w236:string)  [unwired: 14 in]
      }
      frame Default {
        w249 = 42 items=["No error", "Argument error", "Memory is full", "Out of zone", "End of file", "File already open", "Generic file I/O error", "File not found", "File permission error", "Disk is full", "Duplicate path", "Too many files open", "System feature not enabled", "Resource file not found", "Cannot add resource", "Resource not found", "Image not found", "Image memory error", "Pen does not exist", "Config type invalid", "Config token not found", "Config parse error", "Config memory error", "Bad external code format", "Bad external code offset", "External code not present", "Null window", "Destroy window error", "Null menu", "Print aborted", "Bad print record", "Print driver error", "Windows error during printing", "Memory error during printing", "Print dialog error", "Generic print error", "Invalid device refnum", "Device not found", "Device parameter error", "Device unit error", "Cannot open device", "Device call aborted", "Generic error", "Cancelled by user", "Object ID too low", "Object ID too high", "Object not in heap", "Unknown heap", "Unknown object (invalid DefProc)", "Unknown object (DefProc not in table)", "Message out of range", "Invalid (null) method", "Unknown message", "Manager call not supported", "Bad address", "Network operation in progress", "Network operation timed out", "Connection is busy", "Network attribute not supported", "Network error", "Address in use", "System out of memory", "Connection aborted", "Connection refused", "Not connected", "Already connected", "Connection closed", "Initialization error (interapplication manager)", "Bad occurrence", "Wait on unbound occurrence handler", "Occurrence queue overflow", "Datalog type conflict", "Unused", "Unrecognized type (interapplication manager)", "Memory corrupt", "Failed to make temporary DLL", "Old CIN version", "Drag socket not found", "Failed to load drop-object", "Failed to register OLE object", "Failed to release OLE object", "Format specifier type mismatch", "Unknown format specifier", "Too few format specifiers", "Too many format specifiers", "Scan failed", "Newer CIN version", "Error converting to variant", "Runtime menu error", "Password tampered", "Variant attribute not found", "Incompatible variant data type", "Event data is not available", "Event Store is not present", "Occurrence is not found", "Event Queue is not created", "Event info is not available", "Refnum passed is NULL", "Error retrieving Class GUID", "Error retrieving CoClass GUID", "Error retrieving TypeLib GUID.", "Bad built application magic bytes.", "Specific driver is different from the specific driver associated with the Logical Name.", "There is no session opened to the class driver.", "Max Error", "MAX - Error with config objects", "MAX - Error loading configuration", "MAX - Group not supported"]
        # "Current State"
        n146 = Format Into String(format string="Software Exception: Unhandled State \"%s\"." ("message"), error in=w245, w240) -> (resulting string=w248:string, error out=w247:errorcluster)  [unwired: 1 in]
        n147 = call <vilib>:"Error Cluster From Error Code.vi"("show call chain? (False)"=TRUE, "error in (no error)"=w247, "error message (\"\")"=w248, "error code (0)"=w249) -> ("error out"=w246:errorcluster)  [unwired: 5 in]
        n148 = call <vilib>:"Add State(s) to Queue__jki_lib_state_machine.vi"("State(s) in (\"\")"=w244) -> ("States Out"=w243:string)  [unwired: 14 in]
      }
      frame "Initialize Core Data" {
        # "originally closed?"
        # "exe?"
        n149 = property class="VI"() -> ("Front Panel.Open"=w260:bool)  [unwired: 2 in, 2 out]
        n150 = property class="App"() -> ("App.Kind"=w259:T4)  [unwired: 2 in, 2 out]
        n151 = control-ref of="Current VI Reference"() -> (w253:refnum<vi>)
        n152 = Not(x=w260) -> (.not. x?=w257:bool)
        n153 = Equal?(x=w259, y=T4."Run Time System" ("Application:Kind")) -> (x = y?=w256:bool)
        n154 = Or(x=w257, y=w256) -> (x .or. y?=w254:bool)
        n155 = Bundle By Name(cluster=w255, "Core.Current VI Reference"=w253, "Core.Close Panel on Exit?"=w254) -> (w262:T7)
        n156 = call <vilib>:"Add State(s) to Queue__jki_lib_state_machine.vi"("State(s) in (\"\")"=w264) -> ("States Out"=w263:string)  [unwired: 14 in]
      }
      frame "Error Handler" {
        n157 = call <vilib>:"General Error Handler.vi"("error in (no error)"=w268) -> ()  [unwired: 10 in, 5 out]
        n158 = call <vilib>:"Add State(s) to Queue__jki_lib_state_machine.vi"("State(s) in Front (\"\")"="/* Post Error States", "State(s) in (\"\")"=w272) -> ("States Out"=w271:string)  [unwired: 13 in]
      }
      frame "Exit" {
        n159 = call <vilib>:"Add State(s) to Queue__jki_lib_state_machine.vi"("State(s) in (\"\")"=w279) -> ("States Out"=w278:string)  [unwired: 14 in]
        n160 = Quit LabVIEW() -> ()  [unwired: 1 in]
      }
      frame "--------- Library --------" {
        n161 = call <vilib>:"Add State(s) to Queue__jki_lib_state_machine.vi"("State(s) in (\"\")"=w285) -> ("States Out"=w284:string)  [unwired: 14 in]
      }
      frame "S7: Initialize" {
        n162 = property on="PLC" class="Bool (严格)"("Val(Sgnl)"=FALSE ("值(信号)")) -> ()  [unwired: 2 in, 2 out]
      }
      frame "S7: Stop" {
        n163 = call "Stop Module.vi"("error in (no error)"=w294) -> ("error out"=w293:errorcluster)  [unwired: 10 in]
        n164 = call <vilib>:"Add State(s) to Queue__jki_lib_state_machine.vi"("State(s) in (\"\")"=w295) -> ("States Out"=w296:string)  [unwired: 14 in]
      }
      frame "CAN: Start" {
        n165 = while {
          stop <- w307 stop-if-true
          n166 = vi-ref "CAN.vi"() -> (w310:refnum<vi>)
          n167 = call "CallVI.vi"("VI引用"=w310, "状态"=T2."Hidden") -> ("VI引用输出"=w306:refnum<vi>, "错误输出"=w308:errorcluster)  [unwired: 11 in, 1 out]
          n168 = property class="VI"(reference=w306, error in=w308) -> ("Exec.State"=w309:T8)  [unwired: 2 out]
          n169 = case shown="\"Running\"" w309 {
            tunnel: [w311 TRUE TRUE] -> w307
            frame "Bad", Default {
              n170 = Two Button Dialog(message="CAN卡打开失败！" ("消息"), 1:"重试" ("F按钮名称（“取消”）"), 2:"忽略" ("T按钮名称（“确定”）")) -> (T button?=w311:bool)
            }
            frame "Run top level" {
            }
            frame "Running" {
            }
          }
        }
        n171 = call <vilib>:"Add State(s) to Queue__jki_lib_state_machine.vi"("State(s) in (\"\")"=w301) -> ("States Out"=w302:string)  [unwired: 14 in]
      }
      frame "CAN: Stop" {
        n172 = vi-ref "CAN.vi"() -> (w319:refnum<vi>)
        n173 = invoke class="VI" method="Ctrl Val.Set"(reference=w319, "Control Name"="Stop" ("控件名"), "Value"=TRUE) -> ()  [unwired: 2 in, 5 out]
        n174 = call <vilib>:"Add State(s) to Queue__jki_lib_state_machine.vi"("State(s) in (\"\")"=w322) -> ("States Out"=w323:string)  [unwired: 14 in]
      }
      frame "---------- Data ----------" {
        n175 = call <vilib>:"Add State(s) to Queue__jki_lib_state_machine.vi"("State(s) in (\"\")"=w331) -> ("States Out"=w330:string)  [unwired: 14 in]
      }
      frame "Data: Initialize" {
        w336 = T9 {"Current VI Reference"=refnum, "Close Panel on Exit?"=FALSE}  # Core
        w338 = TRUE  # Your Boolean data
        w337 = ""  # Your string data
        n176 = global write "Global.vi" "程序关闭"(FALSE ("程序关闭")) -> ()
        n177 = global write "Global.vi" "计时开始"(FALSE ("计时结束")) -> ()
        n178 = Bundle("Core"=w336, "Your Boolean data"=w338, "Your string data"=w337) -> (w340:T7)  [unwired: 1 in]
        n179 = call <vilib>:"Add State(s) to Queue__jki_lib_state_machine.vi"("State(s) in (\"\")"=w342) -> ("States Out"=w341:string)  [unwired: 14 in]
      }
      frame "Data: Cleanup" {
        n180 = Unbundle By Name(w345) -> ("Core.Current VI Reference"=w348:refnum<vi>)
        n181 = Close Reference(reference=w348, error in (no error)=w347) -> (error out=w346:errorcluster)
        n182 = call <vilib>:"Add State(s) to Queue__jki_lib_state_machine.vi"("State(s) in (\"\")"=w350) -> ("States Out"=w349:string)  [unwired: 14 in]
      }
      frame "---------- UI ----------" {
        # "Do not put any code in this frame.\n(It is a separator no-op. You can make a copy of this frame to create a new UI frame)"
        n183 = call <vilib>:"Add State(s) to Queue__jki_lib_state_machine.vi"("State(s) in (\"\")"=w356) -> ("States Out"=w355:string)  [unwired: 14 in]
      }
      frame "UI: Initialize" {
        n184 = disable-structure shown="禁用" {
          frame Disabled {
            n185 = vi-ref "Auto.vi"() -> (w366:refnum<vi>)
            n186 = invoke class="VI" method="Ctrl Val.Set"(reference=w366, "Control Name"="STEP" ("控件名"), "Value"="进入自动" ("控件名")) -> ()  [unwired: 2 in, 5 out]
          }
          frame Enabled {
          }
        }
        n187 = disable-structure shown="启用" {
          disable-tunnel: [w373 _] -> w360
          disable-tunnel: w357 -> [w372 _]
          frame Enabled {
            n188 = vi-ref "A170316-11_Auto.vi"() -> (w367:refnum<vi>)
            n189 = property class="VI"(reference=w367) -> (reference out=w371:refnum<vi>, "FP.State"=w370:T2)  [unwired: 1 in, 1 out]
            n190 = case shown="\"Standard\", 默认" w370 {
              tunnel: w372 -> [w379 w381]
              tunnel: w371 -> [w380 w382]
              tunnel: [w378 w382] -> w368
              tunnel: [w377 w381] -> w369
              frame "Standard", Default {
                n191 = invoke class="VI" method="FP.Close"(reference=w380, error in=w379) -> (reference out=w378:refnum<vi>, error out=w377:errorcluster)  [unwired: 1 in, 1 out]
              }
              frame "Invalid", "Closed" {
              }
            }
            n192 = invoke on="子面板" class="SubPnl" method="Insert VI"(error in=w369, "VI Ref"=w368) -> (error out=w376:errorcluster)  [unwired: 2 in, 3 out]
            n193 = invoke class="VI" method="Run VI"(reference=w368, error in=w376, "Wait until done"=FALSE ("结束前等待"), "Auto Dispose Ref"=TRUE ("自动销毁引用")) -> (error out=w373:errorcluster)  [unwired: 1 in, 4 out]
          }
          frame Disabled {
            n194 = vi-ref "Auto.vi"() -> (w384:refnum<vi>)
            n195 = call "CallVI.vi"("VI引用"=w384, "状态"=T2."Maximized") -> ()  [unwired: 11 in, 3 out]
          }
        }
        n196 = call <vilib>:"Add State(s) to Queue__jki_lib_state_machine.vi"("State(s) in (\"\")"=w363) -> ("States Out"=w362:string)  [unwired: 14 in]
      }
      frame "UI: Init" {
        n197 = stacked-sequence {
          tunnel: w386 -> [_ _ _ _]
          frame #0 {
            w391 = "" ("产品型号")
            n198 = vi-ref "状态读取.vi"() -> (w394:refnum<vi>)
            n199 = global write "Global.vi" "程序关闭"(FALSE ("程序关闭")) -> ()
            n200 = call "CallVI.vi"("VI引用"=w394, "状态"=T2."Hidden") -> ()  [unwired: 11 in, 3 out]
            n201 = local write "产品型号"(w391) -> ()
            n202 = local write "管柱码"(w391) -> ()
            n203 = control-ref of="上序状态"() -> (w392:refnum<vi>)
            n204 = control-ref of="结果显示:"() -> (w393:refnum<vi>)
            n205 = global write "Global.vi" "结果显示"(w393) -> ()
            n206 = global write "Global.vi" "前序显示字"(w392) -> ()
          }
          frame #1 {
            w397 = 0
            n207 = global read "Global.vi" "前序显示字"() -> (w398:refnum<vi>)
            n208 = global write "Global.vi" "合格数量 2"(w397) -> ()
            n209 = global write "Global.vi" "生产数量 2"(w397) -> ()
            n210 = global read "Global1.vi" "用户信息"() -> (w400:T6)
            n211 = global read "Global1.vi" "联机模式"() -> (w399:enum16{"单机", "联网"})
            n212 = property class="Str"(reference=w398, "Value"="" ("值")) -> ()  [unwired: 1 in, 2 out]
            n213 = Unbundle By Name(w400) -> ("用户名"=→"userName":string, "用户权限"=→"userStatus":string)
            n214 = case shown="\"联网\"" w399 {
              tunnel: ["联网" ("connectionMode") "单机" ("connectionMode")] -> w404
              frame "联网" {
              }
              frame "单机", Default {
              }
            }
            "connectionMode" <- w404
          }
          frame #2 {
            n215 = control-ref of="提示信息"() -> (w409:refnum<vi>)
            n216 = control-ref of="自动"() -> (w408:refnum<vi>)
            n217 = control-ref of="VI引用句柄"() -> (w407:refnum<vi>)
            n218 = control-ref of="错误"() -> (w410:refnum<vi>)
            n219 = control-ref of="Result"() -> (w411:refnum<vi>)
            n220 = global write "Global.vi" "提示信息"(w409) -> ()
            n221 = global write "Global.vi" "程序自动"(w408) -> ()
            n222 = global write "Global.vi" "报警图标"(w410) -> ()
            n223 = global write "Global.vi" "Result"(w411) -> ()
            n224 = global write "Global.vi" "更换型号"(w407) -> ()
          }
          frame #3 {
            n225 = call "Start_Client.vi"() -> ()  [unwired: 12 in]
          }
        }
        n226 = call <vilib>:"Add State(s) to Queue__jki_lib_state_machine.vi"("State(s) in (\"\")"=w390) -> ("States Out"=w389:string)  [unwired: 14 in]
      }
      frame "UI: Config" {
        n227 = vi-ref "A170316-11_config.vi"() -> (w413:refnum<vi>)
        n228 = call "CallVI.vi"("VI引用"=w413, "状态"=T2."Standard") -> ()  [unwired: 11 in, 3 out]
        n229 = call <vilib>:"Add State(s) to Queue__jki_lib_state_machine.vi"("State(s) in (\"\")"=w419) -> ("States Out"=w418:string)  [unwired: 14 in]
      }
      frame "UI: Cursor Set" {
        # "Argument"
        n230 = case shown="\"Idle\", 默认" w422 {
          tunnel: w424 -> [w429 w431]
          tunnel: [w428 w430] -> w423
          frame "Idle", Default {
            n231 = call <vilib>:"Unset Busy.vi"("error in (no error)"=w429) -> ("error out"=w428:errorcluster)  [unwired: 10 in]
          }
          frame "Busy" {
            n232 = call <vilib>:"Set Busy.vi"("error in (no error)"=w431) -> ("error out"=w430:errorcluster)  [unwired: 9 in, 1 out]
          }
        }
        n233 = call <vilib>:"Add State(s) to Queue__jki_lib_state_machine.vi"("State(s) in (\"\")"=w427) -> ("States Out"=w426:string)  [unwired: 14 in]
      }
      frame "UI: Front Panel State" {
        # "Argument"
        n234 = Unbundle By Name(w436) -> ("Core.Current VI Reference"=w435:refnum<vi>)
        n235 = case shown="\"Open\", 默认" w434 {
          tunnel: w438 -> [w444 w457]
          tunnel: [w446 w458] -> w437
          tunnel: w435 -> [w445 w455]
          frame "Open", Default {
            n236 = property class="VI"(reference=w445, error in=w444) -> (reference out=w442:refnum<vi>, error out=w443:errorcluster, "Front Panel.Open"=w441:bool)
            n237 = case shown="假" w441 {
              tunnel: [w449 w452] -> w446
              tunnel: w443 -> [w448 w452]
              tunnel: w442 -> [w447 _]
              frame False {
                n238 = invoke class="VI" method="FP.Open"(reference=w447, error in=w448, "Activate"=TRUE, "State"=T2."Standard") -> (error out=w449:errorcluster)  [unwired: 1 in, 4 out]
              }
              frame True {
              }
            }
          }
          frame "Close" {
            n239 = property class="VI"(reference=w455, error in=w457) -> (reference out=w454:refnum<vi>, error out=w456:errorcluster, "Front Panel.Open"=w453:bool)
            n240 = case shown="真" w453 {
              tunnel: [w459 w462] -> w458
              tunnel: w456 -> [w459 w461]
              tunnel: w454 -> [_ w460]
              frame False {
              }
              frame True {
                n241 = invoke class="VI" method="FP.Close"(reference=w460, error in=w461) -> (error out=w462:errorcluster)  [unwired: 1 in, 2 out]
              }
            }
          }
        }
        n242 = call <vilib>:"Add State(s) to Queue__jki_lib_state_machine.vi"("State(s) in (\"\")"=w440) -> ("States Out"=w439:string)  [unwired: 14 in]
      }
      frame "---------- Macro ----------" {
        n243 = call <vilib>:"Add State(s) to Queue__jki_lib_state_machine.vi"("State(s) in (\"\")"=w468) -> ("States Out"=w467:string)  [unwired: 14 in]
      }
      frame "Macro: Initialize" {
        n244 = call <vilib>:"Add State(s) to Queue__jki_lib_state_machine.vi"("State(s) in Front (\"\")"="Data: Initialize\nInitialize Core Data\nS7: Initialize\nIdle\nUI: Init\nUI: Front Panel State >> Open\nUI: Initialize\nUI: Config", "State(s) in (\"\")"=w475) -> ("States Out"=w474:string)  [unwired: 13 in]
      }
      frame "Macro: Exit" {
        n245 = Unbundle By Name(w489) -> ("Core.Close Panel on Exit?"=w488:bool)
        n246 = vi-ref "client.vi"() -> (w477:refnum<vi>)
        n247 = invoke class="VI" method="Abort VI"(reference=w477) -> (reference out=w478:refnum<vi>, error out=w476:errorcluster)  [unwired: 2 in, 1 out]
        n248 = invoke class="VI" method="FP.Close"(reference=w478, error in=w476) -> (reference out=w480:refnum<vi>, error out=w479:errorcluster)  [unwired: 1 in, 1 out]
        n249 = Select(t="UI: Front Panel State >> Close", s=w488, f="") -> (s? t:f=w485:string)
        n250 = Close Reference(reference=w480, error in (no error)=w479) -> ()  [unwired: 1 out]
        n251 = call <vilib>:"Add State(s) to Queue__jki_lib_state_machine.vi"("State(s) in (\"\")"=w485, "State(s) at Back (\"\")"="Data: Cleanup\nExit") -> ("States Out"=w483:string)  [unwired: 13 in]
        n252 = call <vilib>:"Add State(s) to Queue__jki_lib_state_machine.vi"("State(s) in Front (\"\")"=w483, "State(s) in (\"\")"=w492) -> ("States Out"=w491:string)  [unwired: 13 in]
      }
    }
  }
  n253 = call-dynamic "Cleanup.vi"("MenuStrip in"=w6) -> ()  [unwired: 10 in, 1 out]
